vi "FlexMag - 24-03-2023.vi"() -> ()   [LabVIEW 2018] (continued)
                        n8556 = stacked-sequence {
                          frame #0 {
                            n8557 = while {
                              i -> [w14114]
                              stop <- w14115 stop-if-true
                              n8558 = Greater Or Equal?(x=w14114, y=1500) -> (x >= y?=w14112:bool)
                              n8559 = case shown="True" w14112 {
                                frame False {
                                }
                                frame True {
                                n8560 = local write "Warning Message"("Transfer process canceled!\nCH2 Left Slow Sensor problem" ("Warning Message")) -> ()
                                n8561 = local write "trns error"(TRUE ("TRNS error")) -> ()
                                }
                              }
                              n8562 = local read "CH2_Left_Slow_DI"() -> (w14110:bool)
                              n8563 = case shown="False" w14110 {
                                tunnel: [FALSE ("CH1_Trns_BP_Left_DO") TRUE ("CH1_Trns_BP_Left_DO")] -> w14111
                                frame False {
                                n8564 = Wait Until Next ms Multiple(millisecond multiple=u32 200) -> ()  [unwired: 1 out]
                                }
                                frame True {
                                }
                              }
                              n8565 = local read "ch1-2 transfer"() -> (w14118:bool)
                              n8566 = local read "ABORT"() -> (w14117:bool)
                              n8567 = Not(x=w14118) -> (.not. x?=w14116:bool)
                              n8568 = Compound Arithmetic op=OR(w14111, w14117, w14116) -> (w14115:bool)
                            }
                          }
                          frame #1 {
                            n8569 = flat-sequence {
                              frame #0 {
                                n8570 = local read "Cst_Speed_Low"() -> (w14124:dbl)
                                n8571 = local write "Cassette_Servo_Speed AO"(w14124) -> ()
                                n8572 = Wait (ms)(milliseconds to wait=u32 100) -> ()  [unwired: 1 out]
                              }
                              frame #1 {
                                n8573 = local write "Cassette_Servo_Speed Set"(TRUE ("Cassette_Servo_Speed Set")) -> ()
                              }
                              frame #2 {
                                n8574 = Wait (ms)(milliseconds to wait=u32 100) -> ()  [unwired: 1 out]
                              }
                            }
                          }
                          frame #2 {
                            n8575 = while {
                              i -> [w14131]
                              stop <- w14132 stop-if-true
                              n8576 = Greater Or Equal?(x=w14131, y=100) -> (x >= y?=w14129:bool)
                              n8577 = case shown="True" w14129 {
                                frame False {
                                }
                                frame True {
                                n8578 = local write "Warning Message"("Transfer process canceled!\nLeft Slow Sensor problem" ("Warning Message")) -> ()
                                n8579 = local write "trns error"(TRUE ("TRNS error")) -> ()
                                }
                              }
                              n8580 = disable-structure shown="Enabled" {
                                disable-tunnel: [w14137 w14143] -> w14128
                                frame Disabled {
                                n8581 = local read "Cnt_Left_Slow DI"() -> (w14136:bool)
                                n8582 = case shown="False" w14136 {
                                tunnel: [FALSE ("CH1_Trns_BP_Left_DO") TRUE ("CH1_Trns_BP_Left_DO")] -> w14137
                                frame False {
                                n8583 = Wait Until Next ms Multiple(millisecond multiple=u32 200) -> ()  [unwired: 1 out]
                                n8584 = local write "Cnt_Left_Slow DO"(TRUE ("TRNS error")) -> ()
                                }
                                frame True {
                                }
                                }
                                }
                                frame Enabled {
                                n8585 = local read "CH2_Left_Slow_DI"() -> (w14142:bool)
                                n8586 = case shown="True" w14142 {
                                tunnel: [TRUE ("TRNS error") FALSE ("TRNS error")] -> w14143
                                frame False {
                                }
                                frame True {
                                n8587 = local write "CH2_Left_Slow_DO"(TRUE ("CH2_Left_Slow_DO")) -> ()
                                n8588 = Wait Until Next ms Multiple(millisecond multiple=u32 200) -> ()  [unwired: 1 out]
                                }
                                }
                                }
                              }
                              n8589 = local read "ch1-2 transfer"() -> (w14135:bool)
                              n8590 = local read "ABORT"() -> (w14134:bool)
                              n8591 = Not(x=w14135) -> (.not. x?=w14133:bool)
                              n8592 = Compound Arithmetic op=OR(w14128, w14134, w14133) -> (w14132:bool)
                            }
                          }
                        }
                      }
                      frame True {
                      }
                    }
                  }
                }
              }
              frame #32 {
                n8593 = local read "ch1-2 transfer"() -> (w14150:bool)
                n8594 = case shown="True" w14150 {
                  frame False {
                  }
                  frame True {
                    n8595 = local read "ABORT"() -> (w14151:bool)
                    n8596 = case shown="False" w14151 {
                      frame False {
                        n8597 = local write "trns 1-2 led 15"(TRUE ("trns 1-2 led 1")) -> ()
                        n8598 = Wait (ms)(milliseconds to wait=u32 100) -> ()  [unwired: 1 out]
                      }
                      frame True {
                      }
                    }
                  }
                }
              }
              frame #33 {
                n8599 = local read "ch1-2 transfer"() -> (w14154:bool)
                n8600 = case shown="True" w14154 {
                  frame False {
                  }
                  frame True {
                    n8601 = local read "ABORT"() -> (w14155:bool)
                    n8602 = case shown="False" w14155 {
                      frame False {
                        n8603 = stacked-sequence {
                          frame #0 {
                            n8604 = while {
                              i -> [w14160]
                              stop <- w14161 stop-if-true
                              n8605 = Greater Or Equal?(x=w14160, y=600) -> (x >= y?=w14158:bool)
                              n8606 = case shown="True" w14158 {
                                frame False {
                                }
                                frame True {
                                n8607 = local write "Warning Message"("Transfer process canceled!\nCH2 Left Limit Sensor problem" ("Warning Message")) -> ()
                                n8608 = local write "trns error"(TRUE ("TRNS error")) -> ()
                                }
                              }
                              n8609 = local read "CH2_Left_Limit_DI"() -> (w14156:bool)
                              n8610 = case shown="False" w14156 {
                                tunnel: [FALSE ("CH1_Trns_BP_Left_DO") TRUE ("CH1_Trns_BP_Left_DO")] -> w14157
                                frame False {
                                n8611 = Wait Until Next ms Multiple(millisecond multiple=u32 200) -> ()  [unwired: 1 out]
                                }
                                frame True {
                                }
                              }
                              n8612 = local read "ch1-2 transfer"() -> (w14164:bool)
                              n8613 = local read "ABORT"() -> (w14163:bool)
                              n8614 = Not(x=w14164) -> (.not. x?=w14162:bool)
                              n8615 = Compound Arithmetic op=OR(w14157, w14163, w14162) -> (w14161:bool)
                            }
                          }
                          frame #1 {
                            n8616 = while {
                              i -> [w14174]
                              stop <- w14175 stop-if-true
                              n8617 = Greater Or Equal?(x=w14174, y=100) -> (x >= y?=w14172:bool)
                              n8618 = case shown="True" w14172 {
                                frame False {
                                }
                                frame True {
                                n8619 = local write "Warning Message"("Transfer process canceled!\nCassette Servo couldn't be stopped" ("Warning Message")) -> ()
                                n8620 = local write "trns error"(TRUE ("TRNS error")) -> ()
                                }
                              }
                              n8621 = local read "Casette_Servo_Start/Stop DI"() -> (w14170:bool)
                              n8622 = case shown="True" w14170 {
                                tunnel: [TRUE ("CH1_Trns_BP_Left_DO") FALSE ("CH1_Trns_BP_Left_DO")] -> w14171
                                frame False {
                                }
                                frame True {
                                n8623 = Wait Until Next ms Multiple(millisecond multiple=u32 200) -> ()  [unwired: 1 out]
                                n8624 = local write "Casette_Servo_Start/Stop DO"(FALSE ("TRNS error")) -> ()
                                }
                              }
                              n8625 = local read "ch1-2 transfer"() -> (w14178:bool)
                              n8626 = local read "ABORT"() -> (w14177:bool)
                              n8627 = Not(x=w14178) -> (.not. x?=w14176:bool)
                              n8628 = Compound Arithmetic op=OR(w14171, w14177, w14176) -> (w14175:bool)
                            }
                          }
                          frame #2 {
                            n8629 = flat-sequence {
                              frame #0 {
                                n8630 = local write "Cassette_Servo_Speed AO"(0.0 ("Cassette_Servo_Speed AO")) -> ()
                                n8631 = Wait (ms)(milliseconds to wait=u32 200) -> ()  [unwired: 1 out]
                              }
                              frame #1 {
                                n8632 = local write "Cassette_Servo_Speed Set"(TRUE ("Cassette_Servo_Speed Set")) -> ()
                              }
                            }
                          }
                        }
                      }
                      frame True {
                      }
                    }
                  }
                }
              }
              frame #34 {
                n8633 = local read "ch1-2 transfer"() -> (w14188:bool)
                n8634 = case shown="True" w14188 {
                  frame False {
                  }
                  frame True {
                    n8635 = local read "ABORT"() -> (w14189:bool)
                    n8636 = case shown="False" w14189 {
                      frame False {
                        n8637 = local write "trns 1-2 led 16"(TRUE ("trns 1-2 led 1")) -> ()
                        n8638 = Wait (ms)(milliseconds to wait=u32 100) -> ()  [unwired: 1 out]
                      }
                      frame True {
                      }
                    }
                  }
                }
              }
              frame #35 {
                n8639 = local read "ch1-2 transfer"() -> (w14192:bool)
                n8640 = case shown="True" w14192 {
                  frame False {
                  }
                  frame True {
                    n8641 = local read "ABORT"() -> (w14193:bool)
                    n8642 = case shown="False" w14193 {
                      frame False {
                        n8643 = local read "target chamber"() -> (w14195:dbl)
                        n8644 = Equal?(x=w14195, y=2.0) -> (x = y?=w14196:bool)
                        n8645 = case shown="True" w14196 {
                          frame False {
                          }
                          frame True {
                            n8646 = while {
                              i -> [w14201]
                              stop <- w14202 stop-if-true
                              n8647 = Greater Or Equal?(x=w14201, y=100) -> (x >= y?=w14199:bool)
                              n8648 = case shown="True" w14199 {
                                frame False {
                                }
                                frame True {
                                n8649 = local write "Warning Message"("Transfer process canceled!\nCH2 Cassette Fix problem" ("Warning Message")) -> ()
                                n8650 = local write "trns error"(TRUE ("TRNS error")) -> ()
                                }
                              }
                              n8651 = local read "CH2_Cst_Fix_Down_DI"() -> (w14197:bool)
                              n8652 = case shown="False" w14197 {
                                tunnel: [FALSE ("CH1_Trns_BP_Left_DO") TRUE ("CH1_Trns_BP_Left_DO")] -> w14198
                                frame False {
                                n8653 = Wait Until Next ms Multiple(millisecond multiple=u32 200) -> ()  [unwired: 1 out]
                                n8654 = local write "CH2_Cst_Fix_DO"(TRUE ("TRNS error")) -> ()
                                }
                                frame True {
                                }
                              }
                              n8655 = local read "ch1-2 transfer"() -> (w14205:bool)
                              n8656 = local read "ABORT"() -> (w14204:bool)
                              n8657 = Not(x=w14205) -> (.not. x?=w14203:bool)
                              n8658 = Compound Arithmetic op=OR(w14198, w14204, w14203) -> (w14202:bool)
                            }
                          }
                        }
                      }
                      frame True {
                      }
                    }
                  }
                }
              }
              frame #36 {
                n8659 = local read "ch1-2 transfer"() -> (w14212:bool)
                n8660 = case shown="True" w14212 {
                  frame False {
                  }
                  frame True {
                    n8661 = local read "ABORT"() -> (w14213:bool)
                    n8662 = case shown="False" w14213 {
                      frame False {
                        n8663 = local write "trns 1-2 led 17"(TRUE ("trns 1-2 led 17")) -> ()
                        n8664 = Wait (ms)(milliseconds to wait=u32 100) -> ()  [unwired: 1 out]
                      }
                      frame True {
                      }
                    }
                  }
                }
              }
              frame #37 {
                n8665 = local read "ch1-2 transfer"() -> (w14216:bool)
                n8666 = case shown="True" w14216 {
                  frame False {
                  }
                  frame True {
                    n8667 = local read "ABORT"() -> (w14217:bool)
                    n8668 = case shown="False" w14217 {
                      frame False {
                        n8669 = while {
                          i -> [w14222]
                          stop <- w14223 stop-if-true
                          n8670 = Greater Or Equal?(x=w14222, y=100) -> (x >= y?=w14220:bool)
                          n8671 = case shown="True" w14220 {
                            frame False {
                            }
                            frame True {
                              n8672 = local write "Warning Message"("Transfer process canceled!\nCH1 Trns Bp Left coulnt't be closed" ("Warning Message")) -> ()
                              n8673 = local write "trns error"(TRUE ("TRNS error")) -> ()
                            }
                          }
                          n8674 = local read "CH1_Trns_BP_Left_DI"() -> (w14218:bool)
                          n8675 = case shown="True" w14218 {
                            tunnel: [TRUE ("CH1_Trns_BP_Left_DO") FALSE ("CH1_Trns_BP_Left_DO")] -> w14219
                            frame False {
                            }
                            frame True {
                              n8676 = Wait Until Next ms Multiple(millisecond multiple=u32 200) -> ()  [unwired: 1 out]
                              n8677 = local write "CH1_Trns_BP_Left_DO"(FALSE ("TRNS error")) -> ()
                            }
                          }
                          n8678 = local read "ch1-2 transfer"() -> (w14226:bool)
                          n8679 = local read "ABORT"() -> (w14225:bool)
                          n8680 = Not(x=w14226) -> (.not. x?=w14224:bool)
                          n8681 = Compound Arithmetic op=OR(w14219, w14225, w14224) -> (w14223:bool)
                        }
                      }
                      frame True {
                      }
                    }
                  }
                }
              }
              frame #38 {
                n8682 = local read "ch1-2 transfer"() -> (w14233:bool)
                n8683 = case shown="True" w14233 {
                  frame False {
                  }
                  frame True {
                    n8684 = local read "ABORT"() -> (w14234:bool)
                    n8685 = case shown="False" w14234 {
                      frame False {
                        n8686 = local write "trns 1-2 led 18"(TRUE ("trns 1-2 led 17")) -> ()
                        n8687 = Wait (ms)(milliseconds to wait=u32 100) -> ()  [unwired: 1 out]
                      }
                      frame True {
                      }
                    }
                  }
                }
              }
              frame #39 {
                n8688 = local read "ch1-2 transfer"() -> (w14237:bool)
                n8689 = case shown="True" w14237 {
                  frame False {
                  }
                  frame True {
                    n8690 = local read "ABORT"() -> (w14238:bool)
                    n8691 = case shown="False" w14238 {
                      frame False {
                        n8692 = while {
                          i -> [w14243]
                          stop <- w14244 stop-if-true
                          n8693 = Greater Or Equal?(x=w14243, y=100) -> (x >= y?=w14241:bool)
                          n8694 = case shown="True" w14241 {
                            frame False {
                            }
                            frame True {
                              n8695 = local write "Warning Message"("Transfer process canceled!\nCH2 Trns Bp Right coulnt't be closed" ("Warning Message")) -> ()
                              n8696 = local write "trns error"(TRUE ("TRNS error")) -> ()
                            }
                          }
                          n8697 = local read "CH2_Trns_BP_Right_DI"() -> (w14239:bool)
                          n8698 = case shown="True" w14239 {
                            tunnel: [TRUE ("CH1_Trns_BP_Left_DO") FALSE ("CH1_Trns_BP_Left_DO")] -> w14240
                            frame False {
                            }
                            frame True {
                              n8699 = local write "CH2_Trns_BP_Right_DO"(FALSE ("TRNS error")) -> ()
                              n8700 = Wait Until Next ms Multiple(millisecond multiple=u32 200) -> ()  [unwired: 1 out]
                            }
                          }
                          n8701 = local read "ch1-2 transfer"() -> (w14247:bool)
                          n8702 = local read "ABORT"() -> (w14246:bool)
                          n8703 = Not(x=w14247) -> (.not. x?=w14245:bool)
                          n8704 = Compound Arithmetic op=OR(w14240, w14246, w14245) -> (w14244:bool)
                        }
                      }
                      frame True {
                      }
                    }
                  }
                }
              }
              frame #40 {
                n8705 = local read "ch1-2 transfer"() -> (w14254:bool)
                n8706 = case shown="True" w14254 {
                  frame False {
                  }
                  frame True {
                    n8707 = local read "ABORT"() -> (w14255:bool)
                    n8708 = case shown="False" w14255 {
                      frame False {
                        n8709 = local write "trns 1-2 led 19"(TRUE ("trns 1-2 led 17")) -> ()
                        n8710 = Wait (ms)(milliseconds to wait=u32 100) -> ()  [unwired: 1 out]
                      }
                      frame True {
                      }
                    }
                  }
                }
              }
              frame #41 {
                n8711 = local read "ch1-2 transfer"() -> (w14258:bool)
                n8712 = case shown="True" w14258 {
                  frame False {
                  }
                  frame True {
                    n8713 = local read "ABORT"() -> (w14259:bool)
                    n8714 = case shown="False" w14259 {
                      frame False {
                        n8715 = stacked-sequence {
                          frame #0 {
                            n8716 = local read "ch1-2 transfer"() -> (w14260:bool)
                            n8717 = case shown="True" w14260 {
                              frame False {
                              }
                              frame True {
                                n8718 = local write "CH1_Trns_Gv_Open_DO"(FALSE ("trns clear")) -> ()
                              }
                            }
                          }
                          frame #1 {
                            n8719 = while {
                              i -> [w14266]
                              stop <- w14267 stop-if-true
                              n8720 = Greater Or Equal?(x=w14266, y=600) -> (x >= y?=w14264:bool)
                              n8721 = case shown="True" w14264 {
                                frame False {
                                }
                                frame True {
                                n8722 = local write "Warning Message"("Transfer process canceled!\nCH1-CH2 Trns GV couldn't be closed" ("Warning Message")) -> ()
                                n8723 = local write "trns error"(TRUE ("TRNS error")) -> ()
                                }
                              }
                              n8724 = local read "CH1_Trns_Gv_Close_DI"() -> (w14262:bool)
                              n8725 = case shown="False" w14262 {
                                tunnel: [FALSE ("CH1_Trns_BP_Left_DO") TRUE ("CH1_Trns_BP_Left_DO")] -> w14263
                                frame False {
                                n8726 = local write "CH1_Trns_Gv_Close_DO"(TRUE ("TRNS error")) -> ()
                                n8727 = Wait Until Next ms Multiple(millisecond multiple=u32 200) -> ()  [unwired: 1 out]
                                }
                                frame True {
                                }
                              }
                              n8728 = local read "ch1-2 transfer"() -> (w14270:bool)
                              n8729 = local read "ABORT"() -> (w14269:bool)
                              n8730 = Not(x=w14270) -> (.not. x?=w14268:bool)
                              n8731 = Compound Arithmetic op=OR(w14263, w14269, w14268) -> (w14267:bool)
                            }
                          }
                        }
                      }
                      frame True {
                      }
                    }
                  }
                }
              }
              frame #42 {
                n8732 = local read "ch1-2 transfer"() -> (w14277:bool)
                n8733 = case shown="True" w14277 {
                  frame False {
                  }
                  frame True {
                    n8734 = local read "ABORT"() -> (w14278:bool)
                    n8735 = case shown="False" w14278 {
                      frame False {
                        n8736 = local write "trns 1-2 led 20"(TRUE ("trns 1-2 led 17")) -> ()
                        n8737 = Wait (ms)(milliseconds to wait=u32 100) -> ()  [unwired: 1 out]
                      }
                      frame True {
                      }
                    }
                  }
                }
              }
              frame #43 {
                n8738 = local read "ch1-2 transfer"() -> (w14281:bool)
                n8739 = case shown="True" w14281 {
                  frame False {
                  }
                  frame True {
                    n8740 = local read "ABORT"() -> (w14282:bool)
                    n8741 = case shown="False" w14282 {
                      frame False {
                        n8742 = local read "target chamber"() -> (w14283:dbl)
                        n8743 = Equal?(x=w14283, y=2.0) -> (x = y?=w14284:bool)
                        n8744 = case shown="True" w14284 {
                          frame False {
                          }
                          frame True {
                            n8745 = stacked-sequence {
                              frame #0 {
                                n8746 = local read "ch1-2 transfer"() -> (w14286:bool)
                                n8747 = case shown="True" w14286 {
                                frame False {
                                }
                                frame True {
                                n8748 = local write "CH2_PetCool_Up_DO"(FALSE ("trns clear")) -> ()
                                }
                                }
                              }
                              frame #1 {
                                n8749 = while {
                                i -> [w14292]
                                stop <- w14293 stop-if-true
                                n8750 = Greater Or Equal?(x=w14292, y=300) -> (x >= y?=w14290:bool)
                                n8751 = case shown="True" w14290 {
                                frame False {
                                }
                                frame True {
                                n8752 = local write "Warning Message"("Transfer process canceled!\nCH2 Petcool couldn't be down" ("Warning Message")) -> ()
                                n8753 = local write "trns error"(TRUE ("TRNS error")) -> ()
                                }
                                }
                                n8754 = local read "CH2_PetCool_Down_DI"() -> (w14288:bool)
                                n8755 = case shown="False" w14288 {
                                tunnel: [FALSE ("CH1_Trns_BP_Left_DO") TRUE ("CH1_Trns_BP_Left_DO")] -> w14289
                                frame False {
                                n8756 = local write "CH2_PetCool_Down_DO"(TRUE ("TRNS error")) -> ()
                                n8757 = Wait Until Next ms Multiple(millisecond multiple=u32 200) -> ()  [unwired: 1 out]
                                }
                                frame True {
                                }
                                }
                                n8758 = local read "ch1-2 transfer"() -> (w14296:bool)
                                n8759 = local read "ABORT"() -> (w14295:bool)
                                n8760 = Not(x=w14296) -> (.not. x?=w14294:bool)
                                n8761 = Compound Arithmetic op=OR(w14289, w14295, w14294) -> (w14293:bool)
                                }
                              }
                            }
                          }
                        }
                      }
                      frame True {
                      }
                    }
                  }
                }
              }
              frame #44 {
                n8762 = local read "ch1-2 transfer"() -> (w14303:bool)
                n8763 = case shown="True" w14303 {
                  frame False {
                  }
                  frame True {
                    n8764 = local read "ABORT"() -> (w14304:bool)
                    n8765 = case shown="False" w14304 {
                      frame False {
                        n8766 = local write "trns 1-2 led 21"(TRUE ("trns 1-2 led 17")) -> ()
                        n8767 = Wait (ms)(milliseconds to wait=u32 100) -> ()  [unwired: 1 out]
                      }
                      frame True {
                      }
                    }
                  }
                }
              }
              frame #45 {
                n8768 = local read "ch1-2 transfer"() -> (w14307:bool)
                n8769 = case shown="True" w14307 {
                  frame False {
                  }
                  frame True {
                    n8770 = local read "ABORT"() -> (w14308:bool)
                    n8771 = case shown="False" w14308 {
                      frame False {
                        n8772 = local read "target chamber"() -> (w14310:dbl)
                        n8773 = Equal?(x=w14310, y=2.0) -> (x = y?=w14309:bool)
                        n8774 = case shown="True" w14309 {
                          frame False {
                          }
                          frame True {
                            n8775 = stacked-sequence {
                              frame #0 {
                                n8776 = local read "ch1-2 transfer"() -> (w14312:bool)
                                n8777 = case shown="True" w14312 {
                                frame False {
                                }
                                frame True {
                                n8778 = local write "CH2_SRV1_Piston_Back_DO"(FALSE ("trns clear")) -> ()
                                }
                                }
                              }
                              frame #1 {
                                n8779 = while {
                                i -> [w14318]
                                stop <- w14319 stop-if-true
                                n8780 = Greater Or Equal?(x=w14318, y=200) -> (x >= y?=w14316:bool)
                                n8781 = case shown="True" w14316 {
                                frame False {
                                }
                                frame True {
                                n8782 = local write "Warning Message"("Transfer process canceled!\nCH2 Servo Piston couldn't be forward" ("Warning Message")) -> ()
                                n8783 = local write "trns error"(TRUE ("TRNS error")) -> ()
                                }
                                }
                                n8784 = local read "CH2_SRV1_Piston_For_DI"() -> (w14314:bool)
                                n8785 = case shown="False" w14314 {
                                tunnel: [FALSE ("CH1_Trns_BP_Left_DO") TRUE ("CH1_Trns_BP_Left_DO")] -> w14315
                                frame False {
                                n8786 = local write "CH2_SRV1_Piston_For_DO"(TRUE ("TRNS error")) -> ()
                                n8787 = Wait Until Next ms Multiple(millisecond multiple=u32 200) -> ()  [unwired: 1 out]
                                }
                                frame True {
                                }
                                }
                                n8788 = local read "ch1-2 transfer"() -> (w14322:bool)
                                n8789 = local read "ABORT"() -> (w14321:bool)
                                n8790 = Not(x=w14322) -> (.not. x?=w14320:bool)
                                n8791 = Compound Arithmetic op=OR(w14315, w14321, w14320) -> (w14319:bool)
                                }
                              }
                            }
                          }
                        }
                      }
                      frame True {
                      }
                    }
                  }
                }
              }
              frame #46 {
                n8792 = local read "ch1-2 transfer"() -> (w14329:bool)
                n8793 = case shown="True" w14329 {
                  frame False {
                  }
                  frame True {
                    n8794 = local read "ABORT"() -> (w14330:bool)
                    n8795 = case shown="False" w14330 {
                      frame False {
                        n8796 = local write "trns 1-2 led 22"(TRUE ("trns 1-2 led 17")) -> ()
                        n8797 = Wait (ms)(milliseconds to wait=u32 100) -> ()  [unwired: 1 out]
                      }
                      frame True {
                      }
                    }
                  }
                }
              }
              frame #47 {
                n8798 = local read "ch1-2 transfer"() -> (w14333:bool)
                n8799 = case shown="True" w14333 {
                  frame False {
                  }
                  frame True {
                    n8800 = local read "ABORT"() -> (w14334:bool)
                    n8801 = case shown="False" w14334 {
                      frame False {
                        n8802 = disable-structure shown="Enabled" {
                          frame Disabled {
                            n8803 = stacked-sequence {
                              frame #0 {
                                n8804 = while {
                                i -> [w14339]
                                stop <- w14340 stop-if-true
                                n8805 = Greater Or Equal?(x=w14339, y=100) -> (x >= y?=w14337:bool)
                                n8806 = case shown="True" w14337 {
                                frame False {
                                }
                                frame True {
                                n8807 = local write "Warning Message"("Transfer process canceled!\nRight Slow Sensor problem" ("Warning Message")) -> ()
                                n8808 = local write "trns error"(TRUE ("TRNS error")) -> ()
                                }
                                }
                                n8809 = local read "Cnt_Right_Slow DI"() -> (w14335:bool)
                                n8810 = case shown="True" w14335 {
                                tunnel: [TRUE ("CH1_Trns_BP_Left_DO") FALSE ("CH1_Trns_BP_Left_DO")] -> w14336
                                frame False {
                                }
                                frame True {
                                n8811 = Wait Until Next ms Multiple(millisecond multiple=u32 200) -> ()  [unwired: 1 out]
                                n8812 = local write "Cnt_Right_Slow DO"(FALSE ("TRNS error")) -> ()
                                }
                                }
                                n8813 = local read "ch1-2 transfer"() -> (w14343:bool)
                                n8814 = local read "ABORT"() -> (w14342:bool)
                                n8815 = Not(x=w14343) -> (.not. x?=w14341:bool)
                                n8816 = Compound Arithmetic op=OR(w14336, w14342, w14341) -> (w14340:bool)
                                }
                              }
                              frame #1 {
                                n8817 = while {
                                i -> [w14354]
                                stop <- w14355 stop-if-true
                                n8818 = Greater Or Equal?(x=w14354, y=100) -> (x >= y?=w14352:bool)
                                n8819 = case shown="True" w14352 {
                                frame False {
                                }
                                frame True {
                                n8820 = local write "Warning Message"("Transfer process canceled!\nRight Limit Sensor problem" ("Warning Message")) -> ()
                                n8821 = local write "trns error"(TRUE ("TRNS error")) -> ()
                                }
                                }
                                n8822 = local read "Cnt_Right_Limit DI"() -> (w14350:bool)
                                n8823 = case shown="True" w14350 {
                                tunnel: [TRUE ("CH1_Trns_BP_Left_DO") FALSE ("CH1_Trns_BP_Left_DO")] -> w14351
                                frame False {
                                }
                                frame True {
                                n8824 = Wait Until Next ms Multiple(millisecond multiple=u32 200) -> ()  [unwired: 1 out]
                                n8825 = local write "Cnt_Right_Limit DO"(FALSE ("TRNS error")) -> ()
                                }
                                }
                                n8826 = local read "ch1-2 transfer"() -> (w14358:bool)
                                n8827 = local read "ABORT"() -> (w14357:bool)
                                n8828 = Not(x=w14358) -> (.not. x?=w14356:bool)
                                n8829 = Compound Arithmetic op=OR(w14351, w14357, w14356) -> (w14355:bool)
                                }
                              }
                              frame #2 {
                                n8830 = while {
                                i -> [w14369]
                                stop <- w14370 stop-if-true
                                n8831 = Greater Or Equal?(x=w14369, y=100) -> (x >= y?=w14367:bool)
                                n8832 = case shown="True" w14367 {
                                frame False {
                                }
                                frame True {
                                n8833 = local write "Warning Message"("Transfer process canceled!\nLeft Slow Sensor problem" ("Warning Message")) -> ()
                                n8834 = local write "trns error"(TRUE ("TRNS error")) -> ()
                                }
                                }
                                n8835 = local read "Cnt_Left_Slow DI"() -> (w14365:bool)
                                n8836 = case shown="True" w14365 {
                                tunnel: [TRUE ("CH1_Trns_BP_Left_DO") FALSE ("CH1_Trns_BP_Left_DO")] -> w14366
                                frame False {
                                }
                                frame True {
                                n8837 = Wait Until Next ms Multiple(millisecond multiple=u32 200) -> ()  [unwired: 1 out]
                                n8838 = local write "Cnt_Left_Slow DO"(FALSE ("TRNS error")) -> ()
                                }
                                }
                                n8839 = local read "ch1-2 transfer"() -> (w14373:bool)
                                n8840 = local read "ABORT"() -> (w14372:bool)
                                n8841 = Not(x=w14373) -> (.not. x?=w14371:bool)
                                n8842 = Compound Arithmetic op=OR(w14366, w14372, w14371) -> (w14370:bool)
                                }
                              }
                              frame #3 {
                                n8843 = while {
                                i -> [w14384]
                                stop <- w14385 stop-if-true
                                n8844 = Greater Or Equal?(x=w14384, y=100) -> (x >= y?=w14382:bool)
                                n8845 = case shown="True" w14382 {
                                frame False {
                                }
                                frame True {
                                n8846 = local write "Warning Message"("Transfer process canceled!\nLeft Limit Sensor problem" ("Warning Message")) -> ()
                                n8847 = local write "trns error"(TRUE ("TRNS error")) -> ()
                                }
                                }
                                n8848 = local read "Cnt_Left_Limit DI"() -> (w14380:bool)
                                n8849 = case shown="True" w14380 {
                                tunnel: [TRUE ("CH1_Trns_BP_Left_DO") FALSE ("CH1_Trns_BP_Left_DO")] -> w14381
                                frame False {
                                }
                                frame True {
                                n8850 = Wait Until Next ms Multiple(millisecond multiple=u32 200) -> ()  [unwired: 1 out]
                                n8851 = local write "Cnt_Left_Limit DO"(FALSE ("TRNS error")) -> ()
                                }
                                }
                                n8852 = local read "ch1-2 transfer"() -> (w14388:bool)
                                n8853 = local read "ABORT"() -> (w14387:bool)
                                n8854 = Not(x=w14388) -> (.not. x?=w14386:bool)
                                n8855 = Compound Arithmetic op=OR(w14381, w14387, w14386) -> (w14385:bool)
                                }
                              }
                            }
                          }
                          frame Enabled {
                            w14396 = FALSE ("transfer atm")
                            w14397 = FALSE ("transfer atm")
                            n8856 = local write "CH2_Right_Limit_DO"(w14397) -> ()
                            n8857 = local write "CH2_Right_Slow_DO"(w14397) -> ()
                            n8858 = local write "CH2_Left_Slow_DO"(w14397) -> ()
                            n8859 = local write "CH2_Left_Limit_DO"(w14397) -> ()
                            n8860 = local write "CH1_Right_Limit_DO"(w14397) -> ()
                            n8861 = local write "CH1_Right_Slow_DO"(w14397) -> ()
                            n8862 = Wait (ms)(milliseconds to wait=u32 2000) -> ()  [unwired: 1 out]
                            n8863 = local write "CH3_Right_Limit_DO"(w14396) -> ()
                            n8864 = local write "CH3_Right_Slow_DO"(w14396) -> ()
                            n8865 = local write "CH3_Left_Slow_DO"(w14396) -> ()
                            n8866 = local write "CH3_Left_Limit_DO"(w14396) -> ()
                            n8867 = local write "CH4_Left_Limit_DO"(w14396) -> ()
                            n8868 = local write "CH4_Left_Slow_DO"(w14396) -> ()
                          }
                        }
                      }
                      frame True {
                      }
                    }
                  }
                }
              }
              frame #48 {
                n8869 = local read "ch1-2 transfer"() -> (w14398:bool)
                n8870 = case shown="True" w14398 {
                  frame False {
                  }
                  frame True {
                    n8871 = local read "ABORT"() -> (w14399:bool)
                    n8872 = case shown="False" w14399 {
                      frame False {
                        n8873 = local write "trns 1-2 led 23"(TRUE ("trns 1-2 led 17")) -> ()
                        n8874 = Wait (ms)(milliseconds to wait=u32 100) -> ()  [unwired: 1 out]
                      }
                      frame True {
                      }
                    }
                  }
                }
              }
              frame #49 {
                n8875 = local read "ch1-2 transfer"() -> (w14402:bool)
                n8876 = case shown="True" w14402 {
                  frame False {
                  }
                  frame True {
                    n8877 = local read "ABORT"() -> (w14403:bool)
                    n8878 = case shown="False" w14403 {
                      frame False {
                        n8879 = local write "Buzzer DO"(TRUE ("trns 1-2 led 17")) -> ()
                        n8880 = Wait (ms)(milliseconds to wait=u32 3000) -> ()  [unwired: 1 out]
                        n8881 = local write "System Status"("CH1 to CH2  Transfer Completed" ("System Status")) -> ()
                      }
                      frame True {
                      }
                    }
                  }
                }
              }
              frame #50 {
                n8882 = local read "ch1-2 transfer"() -> (w14407:bool)
                n8883 = case shown="True" w14407 {
                  frame False {
                  }
                  frame True {
                    n8884 = local read "ABORT"() -> (w14408:bool)
                    n8885 = case shown="False" w14408 {
                      frame False {
                        w14409 = u16 2 items=["CH1"=1, "CH2"=2, "CH3"=3, "CH4"=4] ("cassette position selection")
                        w14411 = FALSE ("trns 1-2 led 17")
                        n8886 = Wait (ms)(milliseconds to wait=u32 1000) -> ()  [unwired: 1 out]
                        n8887 = local write "cassette position selection"(w14409) -> ()
                        n8888 = local write "ch1-2 transfer"(FALSE ("trns 1-2 led 17")) -> ()
                        n8889 = local write "Buzzer DO"(FALSE ("trns 1-2 led 17")) -> ()
                        n8890 = local write "System Status"("SEMI-AUTOMATIC MODE " ("System Status")) -> ()
                        n8891 = Not(x=w14411) -> (.not. x?=w14412:bool)
                        n8892 = local write "present location"(2.0 ("present location")) -> ()
                        n8893 = local write "casette_ch1_gui"(w14411) -> ()
                        n8894 = local write "casette_ch2_gui"(w14412) -> ()
                        n8895 = local write "casette_ch3_gui"(w14411) -> ()
                        n8896 = local write "casette_ch4_gui"(w14411) -> ()
                      }
                      frame True {
                      }
                    }
                  }
                }
              }
              frame #51 {
              }
            }
          }
          frame True {
          }
        }
      }
      frame 2 {
        n8897 = local read "ABORT"() -> (w14417:bool)
        n8898 = case shown="False" w14417 {
          frame False {
            n8899 = stacked-sequence {
              frame #0 {
                n8900 = local read "ch2-3 transfer"() -> (w14418:bool)
                n8901 = case shown="True" w14418 {
                  frame False {
                  }
                  frame True {
                    n8902 = local read "present location"() -> (w14421:dbl)
                    n8903 = Wait (ms)(milliseconds to wait=u32 100) -> ()  [unwired: 1 out]
                    n8904 = Equal?(x=w14421, y=2.0) -> (x = y?=w14422:bool)
                    n8905 = case shown="True" w14422 {
                      frame False {
                        n8906 = local write "trns error"(TRUE ("TRNS error")) -> ()
                        n8907 = local write "Warning Message"("Transfer process canceled!\nCassette is not in CH2" ("Warning Message")) -> ()
                      }
                      frame True {
                        n8908 = local write "System Status"("CH2 to CH3  Transfer in Progress" ("System Status")) -> ()
                      }
                    }
                  }
                }
              }
              frame #1 {
                n8909 = local read "ch2-3 transfer"() -> (w14426:bool)
                n8910 = case shown="True" w14426 {
                  frame False {
                  }
                  frame True {
                    n8911 = stacked-sequence {
                      frame #0 {
                        n8912 = local read "ABORT"() -> (w14427:bool)
                        n8913 = case shown="False" w14427 {
                          frame False {
                            n8914 = local write "trns pre check"(TRUE ("trns pre check")) -> ()
                          }
                          frame True {
                          }
                        }
                      }
                      frame #1 {
                        n8915 = Wait (ms)(milliseconds to wait=u32 1000) -> ()  [unwired: 1 out]
                      }
                      frame #2 {
                        n8916 = while {
                          i -> [w14435]
                          stop <- w14432 stop-if-true
                          # "10 min"
                          n8917 = local read "trns pre check"() -> (w14439:bool)
                          n8918 = local read "ch2-3 transfer"() -> (w14431:bool)
                          n8919 = local read "ABORT"() -> (w14433:bool)
                          n8920 = Greater Or Equal?(x=w14435, y=u32 2000 ("millisecond multiple")) -> (x >= y?=w14434:bool)
                          n8921 = Not(x=w14439) -> (.not. x?=w14438:bool)
                          n8922 = Not(x=w14431) -> (.not. x?=w14430:bool)
                          n8923 = Compound Arithmetic op=OR(w14434, w14438, w14433, w14430) -> (w14432:bool)
                          n8924 = Wait Until Next ms Multiple(millisecond multiple=u32 300) -> ()  [unwired: 1 out]
                        }
                      }
                    }
                  }
                }
              }
              frame #2 {
                n8925 = local read "ch2-3 transfer"() -> (w14440:bool)
                n8926 = case shown="True" w14440 {
                  frame False {
                  }
                  frame True {
                    n8927 = local read "trns V?"() -> (w14441:bool)
                    n8928 = case shown="True" w14441 {
                      frame False {
                        n8929 = stacked-sequence {
                          frame #0 {
                            n8930 = local read "ABORT"() -> (w14442:bool)
                            n8931 = case shown="False" w14442 {
                              frame False {
                                w14444 = FALSE ("CH1_CH_ATM_DO")
                                n8932 = local write "CH2_CH_ATM_DO"(w14444) -> ()
                                n8933 = local write "CH3_CH_ATM_DO"(w14444) -> ()
                                n8934 = Wait (ms)(milliseconds to wait=u32 3000) -> ()  [unwired: 1 out]
                              }
                              frame True {
                              }
                            }
                          }
                          frame #1 {
                            n8935 = while {
                              i -> [w14447]
                              stop <- w14448 stop-if-true
                              n8936 = Greater Or Equal?(x=w14447, y=200) -> (x >= y?=w14445:bool)
                              n8937 = case shown="True" w14445 {
                                frame False {
                                }
                                frame True {
                                n8938 = local write "Warning Message"("Transfer process canceled!\nChambers should be on Atmosphere Pressure" ("Warning Message")) -> ()
                                n8939 = local write "trns error"(TRUE ("TRNS error")) -> ()
                                }
                              }
                              n8940 = local read "CH2_CH_ATM_DI"() -> (w14452:bool)
                              n8941 = local read "CH3_CH_ATM_DI"() -> (w14451:bool)
                              n8942 = local read "ch2-3 transfer"() -> (w14454:bool)
                              n8943 = local read "ABORT"() -> (w14455:bool)
                              n8944 = Not(x=w14454) -> (.not. x?=w14453:bool)
                              n8945 = And(x=w14452, y=w14451) -> (x .and. y?=w14450:bool)
                              n8946 = Compound Arithmetic op=OR(w14450, w14455, w14453) -> (w14448:bool)
                              n8947 = Wait Until Next ms Multiple(millisecond multiple=u32 300) -> ()  [unwired: 1 out]
                            }
                          }
                        }
                      }
                      frame True {
                        n8948 = local read "ch2 ch pg torr"() -> (w14464:dbl)
                        n8949 = local read "ch3 ch pg torr"() -> (w14461:dbl)
                        n8950 = Greater Or Equal?(x=w14464, y=0.5) -> (x >= y?=w14460:bool)
                        n8951 = Greater Or Equal?(x=w14461, y=0.5) -> (x >= y?=w14459:bool)
                        n8952 = Or(x=w14460, y=w14459) -> (x .or. y?=w14458:bool)
                        n8953 = local write "trns error"(w14458) -> ()
                      }
                    }
                  }
                }
              }
              frame #3 {
                n8954 = local read "ch2-3 transfer"() -> (w14465:bool)
                n8955 = case shown="True" w14465 {
                  frame False {
                  }
                  frame True {
                    n8956 = local read "ABORT"() -> (w14466:bool)
                    n8957 = case shown="False" w14466 {
                      frame False {
                        n8958 = while {
                          i -> [w14471]
                          stop <- w14472 stop-if-true
                          n8959 = Greater Or Equal?(x=w14471, y=100) -> (x >= y?=w14469:bool)
                          n8960 = case shown="True" w14469 {
                            frame False {
                            }
                            frame True {
                              n8961 = local write "trns error"(TRUE ("TRNS error")) -> ()
                              n8962 = local write "Warning Message"("Transfer process canceled!\nCH2 Trns BP Left couln't be opened" ("Warning Message")) -> ()
                            }
                          }
                          n8963 = local read "CH2_Trns_BP_Left_DI"() -> (w14468:bool)
                          n8964 = case shown="False" w14468 {
                            tunnel: [FALSE ("CH1_Trns_BP_Left_DO") TRUE ("CH1_Trns_BP_Left_DO")] -> w14467
                            frame False {
                              n8965 = Wait Until Next ms Multiple(millisecond multiple=u32 200) -> ()  [unwired: 1 out]
                              n8966 = local write "CH2_Trns_BP_Left_DO"(TRUE ("CH1_Trns_BP_Left_DO")) -> ()
                            }
                            frame True {
                            }
                          }
                          n8967 = local read "ch2-3 transfer"() -> (w14475:bool)
                          n8968 = local read "ABORT"() -> (w14474:bool)
                          n8969 = Not(x=w14475) -> (.not. x?=w14473:bool)
                          n8970 = Compound Arithmetic op=OR(w14467, w14474, w14473) -> (w14472:bool)
                        }
                      }
                      frame True {
                      }
                    }
                  }
                }
              }
              frame #4 {
                n8971 = local read "ch2-3 transfer"() -> (w14482:bool)
                n8972 = case shown="True" w14482 {
                  frame False {
                  }
                  frame True {
                    n8973 = local read "ABORT"() -> (w14483:bool)
                    n8974 = case shown="False" w14483 {
                      frame False {
                        n8975 = local write "trns 2-3 led 1"(TRUE ("trns 1-2 led 1")) -> ()
                        n8976 = Wait (ms)(milliseconds to wait=u32 100) -> ()  [unwired: 1 out]
                      }
                      frame True {
                      }
                    }
                  }
                }
              }
              frame #5 {
                n8977 = local read "ch2-3 transfer"() -> (w14486:bool)
                n8978 = case shown="True" w14486 {
                  frame False {
                  }
                  frame True {
                    n8979 = local read "ABORT"() -> (w14487:bool)
                    n8980 = case shown="False" w14487 {
                      frame False {
                        n8981 = while {
                          i -> [w14492]
                          stop <- w14493 stop-if-true
                          n8982 = Greater Or Equal?(x=w14492, y=100) -> (x >= y?=w14490:bool)
                          n8983 = case shown="True" w14490 {
                            frame False {
                            }
                            frame True {
                              n8984 = local write "trns error"(TRUE ("TRNS error")) -> ()
                              n8985 = local write "Warning Message"("Transfer process canceled!\nCH3 Trns BP Right couln't be opened" ("Warning Message")) -> ()